vi "Controle_Manip_Main_GUI_Backup2.vi"() -> ()   [LabVIEW 2019] (continued)
                    n3203 = local write "Photodiode error out"(w3898) -> ()
                  }
                }
              }
            }
          }
          event "RotStage Exc Home", "RotStage Det Home", "Newport Linear Translation Stage Home": Mouse Down {
            n3204 = event-data() -> ("CtlRef"=w3923:refnum<vi>)  [unwired: 1 in, 7 out]
            n3205 = property class="Bool (strict)"(reference=w3923) -> ("Label.Text"=w3922:string)  [unwired: 1 in, 2 out]
            n3206 = case shown="\"Newport Linear Translation Stage Home\"" w3922 {
              tunnel: 0.0 -> [w3924 w3925 w3926]
              frame "RotStage Det Home", Default {
                n3207 = property on="RotStage Det Angle (°)" class="DigNum (strict)"("Val(Sgnl)"=w3924) -> ()  [unwired: 2 in, 2 out]
              }
              frame "Newport Linear Translation Stage Home" {
                n3208 = property on="Newport Linear Translation Stage Position (mm)" class="DigNum (strict)"("Val(Sgnl)"=w3925) -> ()  [unwired: 2 in, 2 out]
              }
              frame "RotStage Exc Home" {
                n3209 = property on="RotStage Exc Angle (°)" class="DigNum (strict)"("Val(Sgnl)"=w3926) -> ()  [unwired: 2 in, 2 out]
              }
            }
          }
          event "RotStage Exc Jog Backward", "RotStage Det Jog Backward", "RotStage Exc Jog Forward", "RotStage Det Jog Forward", "Newport Linear Translation Stage Jog Forward", "Newport Linear Translation Stage Jog Backward", "PZC Jog Forward", "PZC Jog Backward": Mouse Down {
            n3210 = event-data() -> ("CtlRef"=w3929:refnum<vi>)  [unwired: 1 in, 7 out]
            n3211 = property class="Bool (strict)"(reference=w3929) -> ("Label.Text"=w3927:string, "Value"=w3928:bool)  [unwired: 1 in, 2 out]
            n3212 = case shown="\"PZC Jog Backward\"" w3927 {
              tunnel: w3928 -> [_ _ _ _ _ _ _ _ _]
              frame "RotStage Det Jog Backward" {
                n3213 = local read "RotStage Det Angle Readout (°)"() -> (w3932:dbl)
                n3214 = local read "RotStage Det Angle Step (°)"() -> (w3931:dbl)
                n3215 = Subtract(x=w3932, y=w3931) -> (x-y=w3930:dbl)
                n3216 = property on="RotStage Det Angle (°)" class="DigNum (strict)"("Val(Sgnl)"=w3930) -> ()  [unwired: 2 in, 2 out]
              }
              frame "RotStage Det Jog Forward" {
                n3217 = local read "RotStage Det Angle Readout (°)"() -> (w3934:dbl)
                n3218 = local read "RotStage Det Angle Step (°)"() -> (w3935:dbl)
                n3219 = Add(x=w3934, y=w3935) -> (x+y=w3933:dbl)
                n3220 = property on="RotStage Det Angle (°)" class="DigNum (strict)"("Val(Sgnl)"=w3933) -> ()  [unwired: 2 in, 2 out]
              }
              frame "RotStage Exc Jog Forward" {
                n3221 = local read "RotStage Exc Angle Readout (°)"() -> (w3938:dbl)
                n3222 = local read "RotStage Exc Angle Step (°)"() -> (w3937:dbl)
                n3223 = Add(x=w3938, y=w3937) -> (x+y=w3936:dbl)
                n3224 = property on="RotStage Exc Angle (°)" class="DigNum (strict)"("Val(Sgnl)"=w3936) -> ()  [unwired: 2 in, 2 out]
              }
              frame "Newport Linear Translation Stage Jog Forward" {
                n3225 = local read "Newport Linear Translation Stage Position Readout (mm)"() -> (w3943:dbl)
                n3226 = local read "Newport Linear Translation Stage Step (mm)"() -> (w3942:dbl)
                n3227 = Add(x=w3943, y=w3942) -> (x+y=w3941:dbl)
                n3228 = property on="Newport Linear Translation Stage Position Readout (mm)" class="DigNum (strict)"() -> ("Maximum"=w3939:dbl)  [unwired: 2 in, 2 out]
                n3229 = Less Or Equal?(x=w3941, y=w3939) -> (x <= y?=w3940:bool)
                n3230 = case shown="True" w3940 {
                  tunnel: w3941 -> [_ w3947]
                  frame False {
                    n3231 = stacked-sequence {
                      frame #0 {
                        n3232 = property on="Newport Linear Translation Stage Position Readout (mm)" class="DigNum (strict)"("Blinking"=TRUE) -> ()  [unwired: 2 in, 2 out]
                      }
                      frame #1 {
                        n3233 = Wait (ms)(milliseconds to wait=u32 500) -> ()  [unwired: 1 out]
                      }
                      frame #2 {
                        n3234 = property on="Newport Linear Translation Stage Position Readout (mm)" class="DigNum (strict)"("Blinking"=FALSE) -> ()  [unwired: 2 in, 2 out]
                      }
                    }
                  }
                  frame True {
                    n3235 = property on="Newport Linear Translation Stage Position (mm)" class="DigNum (strict)"("Val(Sgnl)"=w3947) -> ()  [unwired: 2 in, 2 out]
                  }
                }
              }
              frame "Newport Linear Translation Stage Jog Backward" {
                n3236 = local read "Newport Linear Translation Stage Position Readout (mm)"() -> (w3952:dbl)
                n3237 = local read "Newport Linear Translation Stage Step (mm)"() -> (w3951:dbl)
                n3238 = Subtract(x=w3952, y=w3951) -> (x-y=w3949:dbl)
                n3239 = property on="Newport Linear Translation Stage Position Readout (mm)" class="DigNum (strict)"() -> ("Minimum"=w3948:dbl)  [unwired: 2 in, 2 out]
                n3240 = Greater Or Equal?(x=w3949, y=w3948) -> (x >= y?=w3950:bool)
                n3241 = case shown="False" w3950 {
                  tunnel: w3949 -> [_ w3956]
                  frame False {
                    n3242 = stacked-sequence {
                      frame #0 {
                        n3243 = property on="Newport Linear Translation Stage Position Readout (mm)" class="DigNum (strict)"("Blinking"=TRUE) -> ()  [unwired: 2 in, 2 out]
                      }
                      frame #1 {
                        n3244 = Wait (ms)(milliseconds to wait=u32 500) -> ()  [unwired: 1 out]
                      }
                      frame #2 {
                        n3245 = property on="Newport Linear Translation Stage Position Readout (mm)" class="DigNum (strict)"("Blinking"=FALSE) -> ()  [unwired: 2 in, 2 out]
                      }
                    }
                  }
                  frame True {
                    n3246 = property on="Newport Linear Translation Stage Position (mm)" class="DigNum (strict)"("Val(Sgnl)"=w3956) -> ()  [unwired: 2 in, 2 out]
                  }
                }
              }
              frame "RotStage Exc Jog Backward" {
                n3247 = local read "RotStage Exc Angle Readout (°)"() -> (w3959:dbl)
                n3248 = local read "RotStage Exc Angle Step (°)"() -> (w3958:dbl)
                n3249 = Subtract(x=w3959, y=w3958) -> (x-y=w3957:dbl)
                n3250 = property on="RotStage Exc Angle (°)" class="DigNum (strict)"("Val(Sgnl)"=w3957) -> ()  [unwired: 2 in, 2 out]
              }
              frame "PZC Jog Forward" {
                n3251 = local read "PZC200 Instrument Channel"() -> (w3977:string)
                n3252 = local read "PZC Speed (usteps/s)"() -> (w3968:u16)
                n3253 = Number To Decimal String(number=w3968) -> (decimal integer string=w3970:string)  [unwired: 1 in]
                n3254 = Concatenate Strings("1JA" ("Command"), w3970) -> (w3976:string)
                n3255 = call "SendCommand.vi"("Command"=w3976, "Instrument Channel"=w3977) -> ("error out"=w3974:errorcluster, "Instrument Channel out"=w3975:string)  [unwired: 8 in]
                n3256 = call "ReadCommand.vi"("Disable MAV check (F)"=FALSE, "error in"=w3974, "Instrument Channel"=w3975) -> ("error out"=w3971:errorcluster, "Instrument Channel out"=w3973:string)  [unwired: 6 in, 1 out]
                n3257 = while {
                  shift-right: [w3981] -> w3967
                  shift-left: w3973 -> [w3985]
                  shift-right: [w3979] -> w3966
                  shift-left: w3971 -> [w3980]
                  tunnel: ["1ST"] -> w3965
                  stop <- w3982 continue-if-true
                  n3258 = call "PZCGetPos.vi"("error in"=w3980, "Instrument Channel"=w3985) -> ("Instrument Channel Out"=w3981:string, "Position"=w3984:i32, "error out"=w3979:errorcluster)
                  n3259 = Wait (ms)(milliseconds to wait=u32 150) -> ()  [unwired: 1 out]
                  n3260 = local write "PZC Position Readout (usteps)"(w3984) -> ()
                  n3261 = local read "PZC Jog Forward"() -> (w3982:bool)
                }
                n3262 = call "SendCommand.vi"("error in"=w3966, "Command"=w3965, "Instrument Channel"=w3967) -> ("error out"=w3963:errorcluster, "Instrument Channel out"=w3964:string)  [unwired: 7 in]
                n3263 = call "PZCGetPos.vi"("error in"=w3963, "Instrument Channel"=w3964) -> ("Instrument Channel Out"=w3962:string, "Position"=w3960:i32, "error out"=w3961:errorcluster)
                n3264 = local write "PZC Position Readout (usteps)"(w3960) -> ()
                n3265 = local write "PZC Error"(w3961) -> ()
                n3266 = local write "PZC200 Instrument Channel"(w3962) -> ()
              }
              frame Default {
              }
              frame "PZC Jog Backward" {
                n3267 = local read "PZC Speed (usteps/s)"() -> (w3991:u16)
                n3268 = local read "PZC200 Instrument Channel"() -> (w4003:string)
                n3269 = Number To Decimal String(number=w3991) -> (decimal integer string=w3993:string)  [unwired: 1 in]
                n3270 = Concatenate Strings("1JA-" ("Command"), w3993) -> (w4002:string)
                n3271 = call "SendCommand.vi"("Command"=w4002, "Instrument Channel"=w4003) -> ("error out"=w4000:errorcluster, "Instrument Channel out"=w4001:string)  [unwired: 8 in]
                n3272 = call "ReadCommand.vi"("Disable MAV check (F)"=FALSE, "error in"=w4000, "Instrument Channel"=w4001) -> ("error out"=w3997:errorcluster, "Instrument Channel out"=w3998:string)  [unwired: 6 in, 1 out]
                n3273 = while {
                  shift-right: [w4005] -> w3996
                  shift-left: w3997 -> [w4006]
                  shift-right: [w4007] -> w3995
                  shift-left: w3998 -> [w4011]
                  tunnel: ["1ST"] -> w3994
                  stop <- w4009 continue-if-true
                  n3274 = call "PZCGetPos.vi"("error in"=w4006, "Instrument Channel"=w4011) -> ("Instrument Channel Out"=w4007:string, "Position"=w4010:i32, "error out"=w4005:errorcluster)
                  n3275 = Wait (ms)(milliseconds to wait=u32 150) -> ()  [unwired: 1 out]
                  n3276 = local write "PZC Position Readout (usteps)"(w4010) -> ()
                  n3277 = local read "PZC Jog Backward"() -> (w4009:bool)
                }
                n3278 = call "SendCommand.vi"("error in"=w3996, "Command"=w3994, "Instrument Channel"=w3995) -> ("error out"=w3990:errorcluster, "Instrument Channel out"=w3989:string)  [unwired: 7 in]
                n3279 = call "PZCGetPos.vi"("error in"=w3990, "Instrument Channel"=w3989) -> ("Instrument Channel Out"=w3988:string, "Position"=w3986:i32, "error out"=w3987:errorcluster)
                n3280 = local write "PZC Position Readout (usteps)"(w3986) -> ()
                n3281 = local write "PZC Error"(w3987) -> ()
                n3282 = local write "PZC200 Instrument Channel"(w3988) -> ()
              }
            }
          }
          event "RotStage Exc Velocity (°/s)", "RotStage Det Velocity (°/s)", "Newport Linear Translation Stage Velocity (mm/s)": Value Change {
            n3283 = event-data() -> ("CtlRef"=w4014:refnum<vi>, "NewVal"=w4013:dbl)  [unwired: 1 in, 4 out]
            n3284 = local read "ESP 301 On?"() -> (w4012:bool)
            n3285 = case shown="True" w4012 {
              tunnel: w4014 -> [_ w4021]
              tunnel: w4013 -> [_ w4019]
              frame False {
              }
              frame True {
                n3286 = local read "ESP 301 COM Port"() -> (w4018:refnum<visa-resource-name>)
                n3287 = property class="DigNum (strict)"(reference=w4021) -> ("Label.Text"=w4020:string)  [unwired: 1 in, 2 out]
                n3288 = local read "ESP 301 Error"() -> (w4017:errorcluster)
                n3289 = case shown="\"RotStage Det Velocity (°/s)\"" w4020 {
                  tunnel: w4019 -> [w4025 _ w4030 w4040]
                  tunnel: w4018 -> [w4026 w4029 w4032 w4039]
                  tunnel: w4017 -> [w4027 w4028 w4033 w4038]
                  tunnel: [w4023 w4029 w4035 w4037] -> w4016
                  tunnel: [w4022 w4028 w4034 w4036] -> w4015
                  frame "Newport Linear Translation Stage Velocity (mm/s)" {
                    n3290 = call "Set Velocity.vi"("error in (no error)"=w4027, "Velocity (units/s)"=w4025, "Axis (1)"=1, "VISA resource name"=w4026) -> ("error out"=w4022:errorcluster, "VISA resource name out"=w4023:refnum<visa-resource-name>)  [unwired: 2 in]
                  }
                  frame Default {
                  }
                  frame "RotStage Det Velocity (°/s)" {
                    n3291 = call "Set Velocity.vi"("error in (no error)"=w4033, "Velocity (units/s)"=w4030, "Axis (1)"=2, "VISA resource name"=w4032) -> ("error out"=w4034:errorcluster, "VISA resource name out"=w4035:refnum<visa-resource-name>)  [unwired: 2 in]
                  }
                  frame "RotStage Exc Velocity (°/s)" {
                    n3292 = call "Set Velocity.vi"("error in (no error)"=w4038, "Velocity (units/s)"=w4040, "Axis (1)"=3, "VISA resource name"=w4039) -> ("error out"=w4036:errorcluster, "VISA resource name out"=w4037:refnum<visa-resource-name>)  [unwired: 2 in]
                  }
                }
                n3293 = local write "ESP 301 COM Port"(w4016) -> ()
                n3294 = local write "ESP 301 Error"(w4015) -> ()
              }
            }
          }
          event "Save Spectrum", "Save Spectrum N", "Save XY Map", "Save Polarisation", "Save Contrast", "Save Michelson", "Save Custom Diode Spectrum", "Save fPow", "Save PLE": Value Change {
            n3295 = event-data() -> ("CtlRef"=w4049:refnum<vi>)  [unwired: 1 in, 3 out]
            n3296 = property class="Bool (strict)"(reference=w4049) -> ("Label.Text"=w4048:string)  [unwired: 1 in, 2 out]
            n3297 = stacked-sequence {
              tunnel: w4048 -> [_ w4098 _]
              tunnel: [_ w4095 _] -> w4046
              tunnel: [_ w4097 _] -> w4047
              tunnel: [_ w4092 _] -> w4044
              tunnel: [w4050 _ _] -> w4043
              tunnel: [_ w4093 _] -> w4045
              frame #0 {
                n3298 = local read "Excitation Wavelength (nm)"() -> (w4072:dbl)
                n3299 = local read "Wavelength calibration"() -> (w4073:dbl[])
                n3300 = local read "Center Wavelength (nm)"() -> (w4081:dbl)
                n3301 = local read "Experiment Name With Date"() -> (w4077:string)
                n3302 = local read "Map Marker Y Pos"() -> (w4063:i8)
                n3303 = local read "Scan Y Readout (V)"() -> (w4061:dbl)
                n3304 = local read "Scan X Readout (V)"() -> (w4062:dbl)
                n3305 = local read "Exposure Time (ms)"() -> (w4074:dbl)
                n3306 = local read "Map Marker X Pos"() -> (w4064:i8)
                n3307 = local read "Exposure Time (ms)"() -> (w4078:dbl)
                n3308 = local read "Attocubes On?"() -> (w4068:bool)
                n3309 = local read "Excitation Source"() -> (w4079:enum16{"P", "CW", "SK"})
                n3310 = local read "Temperature (K)"() -> (w4082:dbl)
                n3311 = local read "Excitation Power (uW)"() -> (w4084:dbl)
                n3312 = local read "Comment"() -> (w4083:string)
                n3313 = local read "Acq Mode"() -> (w4076:T3)
                n3314 = local read "Log file"() -> (w4075:string)
                n3315 = case shown="True" w4068 {
                  tunnel: [w4085 w4088] -> w4067
                  tunnel: [w4085 w4087] -> w4066
                  tunnel: [w4085 w4086] -> w4065
                  frame False {
                    w4085 = nan
                  }
                  frame True {
                    n3316 = local read "Att Pos Y"() -> (w4087:dbl)
                    n3317 = local read "Att Pos X"() -> (w4088:dbl)
                    n3318 = local read "Att Pos Z"() -> (w4086:dbl)
                  }
                }
                n3319 = Multiply(x=w4084, y=1000000.0) -> (x*y=w4080:dbl)
                n3320 = local read "LightField On?"() -> (w4070:bool)
                n3321 = Bundle("Att Pos X"=w4067, "Att Pos Y"=w4066, "Att Pos Z"=w4065, "Map Marker X Pos"=w4064, "Map Marker Y Pos"=w4063, "Scan X Readout (V)"=w4062, "Scan Y Readout (V)"=w4061) -> (w4060:T5)  [unwired: 1 in]
                "Location cluster" <- w4060
                n3322 = case shown="False" w4070 {
                  tunnel: ["" w4090] -> w4069
                  frame False {
                  }
                  frame True {
                    n3323 = local read "Grating"() -> (w4090:string)
                  }
                }
                n3324 = Bundle("Sample first cooldown"="Sample first cooldown", "SampleOf"="SampleOf", "Synthesis/Name"="Synthesis/Name", "Synthesis/InjTemp"="Synthesis/InjTemp", "Synthesis/Dilution"="Synthesis/Dilution", "Synthesis/Polymer"="Synthesis/Polymer", "Synthesis/DilutionPolyRatio"="Synthesis/DilutionPolyRatio", "Synthesis/Solvent"="Synthesis/Solvent") -> (w4051:T40)  [unwired: 1 in]
                n3325 = Bundle("Comment"=w4083, "Temperature (K)"=w4082, "Center Wavelength (nm)"=w4081, w4080, "Excitation Source"=w4079, "Exposure Time (ms)"=w4078, "Experiment Name With Date"=w4077, "Acq Mode"=w4076, "Log file"=w4075, "Exposure Time (ms)"=w4074, "Wavelength calibration"=w4073, "Excitation Wavelength (nm)"=w4072, "Grating"=w4069, w4060, w4051) -> (w4050:T41)  [unwired: 1 in]
                "Params Save" <- w4050
              }
              frame #1 {
                n3326 = case shown="\"Save Contrast\"" w4098 {
                  tunnel: [w4102 w4147 w4172 w4196 w4218 w4248 w4271 w4294 w4343] -> w4095
                  tunnel: [w4101 w4145 w4171 w4195 w4217 w4247 w4270 w4293 w4340] -> w4092
                  tunnel: [w4100 w4146 w4170 w4194 w4216 w4246 w4269 w4292 w4334] -> w4096
                  tunnel: [w4099 w4144 w4169 w4193 w4215 w4245 w4268 w4291 w4333] -> w4093
                  frame "Save Spectrum N" {
                    n3327 = local read "Acq Mode"() -> (w4103:T3)
                    n3328 = case shown="\"Spectrum\", Default" w4103 {
                      tunnel: [w4112 w4133] -> w4102
                      tunnel: [w4111 w4132] -> w4101
                      tunnel: [w4105 w4126] -> w4100
                      tunnel: [w4104 w4125] -> w4099
                      frame "Spectrum", Default {
                        w4104 = T42."Time Trace" ("Measurement type")
                        n3329 = invoke on="CCD 2D Image Main" class="IntGraph (strict)" method="Get Image"() -> ("image data"=w4105:T43)  [unwired: 6 in, 5 out]
                        n3330 = local read "BackgroundSpec"() -> (w4109:dbl[])
                        n3331 = local read "Pol in path?"() -> (w4108:bool)
                        n3332 = local read "DotNum"() -> (w4110:dbl)
                        n3333 = local read "Data"() -> (w4118:T26)
                        n3334 = local read "Params Save"() -> (w4121:T4)
                        n3335 = Index Array(array=w4118, index=0) -> (element=w4116:T44)
                        n3336 = case shown="True" w4108 {
                          tunnel: [w4122 w4123] -> w4106
                          tunnel: [w4122 w4124] -> w4107
                          frame False {
                            w4122 = nan
                          }
                          frame True {
                            n3337 = local read "RotStage Exc Angle Readout (°)"() -> (w4124:dbl)
                            n3338 = local read "RotStage Det Angle Readout (°)"() -> (w4123:dbl)
                          }
                        }
                        n3339 = Unbundle By Name(w4116) -> ("Image"=w4115:dbl[][][])
                        "Image" <- w4115
                        n3340 = Index Array(array=w4115, index (dim 1)=0 ("disabled index (row)")) -> (element=w4114:dbl[][])  [unwired: 2 in]
                        n3341 = Build Array(w4107) -> (w4120:dbl[])
                        n3342 = Build Array(w4106) -> (w4119:dbl[])
                        n3343 = call "Format&SaveDataCleanbckp.vi"("Measurement type"=w4104, "Params Save"=w4121, "DotNum"=w4110, "Suppl"=w4109, "Data_CCD_px"=w4114, "L2Exc_deg"=w4120, "L2Det_deg"=w4119) -> ("FullComment"=w4111:string, "WrittenDatasetName"=w4112:string)  [unwired: 9 in, 2 out]
                      }
                      frame "Image" {
                        w4125 = T42."Time Trace" ("Measurement type")
                        n3344 = invoke on="CCD 2D Image Main" class="IntGraph (strict)" method="Get Image"() -> ("image data"=w4126:T43)  [unwired: 6 in, 5 out]
                        n3345 = local read "BackgroundSpec"() -> (w4130:dbl[])
                        n3346 = local read "Pol in path?"() -> (w4129:bool)
                        n3347 = local read "DotNum"() -> (w4131:dbl)
                        n3348 = local read "Data"() -> (w4137:T26)
                        n3349 = local read "Params Save"() -> (w4140:T4)
                        n3350 = case shown="True" w4129 {
                          tunnel: [w4141 w4142] -> w4127
                          tunnel: [w4141 w4143] -> w4128
                          frame False {
                            w4141 = nan
                          }
                          frame True {
                            n3351 = local read "RotStage Exc Angle Readout (°)"() -> (w4143:dbl)
                            n3352 = local read "RotStage Det Angle Readout (°)"() -> (w4142:dbl)
                          }
                        }
                        n3353 = Index Array(array=w4137, index=0) -> (element=w4135:T44)
                        n3354 = Unbundle By Name(w4135) -> ("Image"=w4134:dbl[][][])
                        n3355 = Build Array(w4128) -> (w4139:dbl[])
                        n3356 = Build Array(w4127) -> (w4138:dbl[])
                        n3357 = call "Format&SaveDataCleanbckp.vi"("Measurement type"=w4125, "Params Save"=w4140, "DotNum"=w4131, "Main 3D Data to write"=w4134, "Suppl"=w4130, "L2Exc_deg"=w4139, "L2Det_deg"=w4138) -> ("FullComment"=w4132:string, "WrittenDatasetName"=w4133:string)  [unwired: 9 in, 2 out]
                      }
                    }
                  }
                  frame "Save XY Map" {
                    w4144 = T42."XY Intensity Map" ("Measurement type")
                    n3358 = local read "Pol in path?"() -> (w4158:bool)
                    n3359 = local read "Params Save"() -> (w4165:T4)
                    n3360 = local read "BackgroundSpec"() -> (w4162:dbl[])
                    n3361 = local read "Params XY Map SubVI"() -> (w4155:T23)
                    n3362 = local read "Map Marker Y Pos"() -> (w4153:i8)
                    n3363 = local read "XYMap Data"() -> (w4164:i32[][])
                    n3364 = local read "Map Marker X Pos"() -> (w4154:i8)
                    n3365 = local read "XYPositions"() -> (w4161:dbl[][])
                    n3366 = Format Into String(w4154) -> (resulting string=w4152:string)  [unwired: 3 in, 1 out]
                    n3367 = Format Into String(w4153) -> (resulting string=w4151:string)  [unwired: 3 in, 1 out]
                    n3368 = case shown="True" w4158 {
                      tunnel: [w4166 w4167] -> w4157
                      tunnel: [w4166 w4168] -> w4156
                      frame False {
                        w4166 = nan
                      }
                      frame True {
                        n3369 = local read "RotStage Exc Angle Readout (°)"() -> (w4168:dbl)
                        n3370 = local read "RotStage Det Angle Readout (°)"() -> (w4167:dbl)
                      }
                    }
                    n3371 = Concatenate Strings("\n### Map @ " ("string"), w4152, "x" ("string"), w4151) -> (w4150:string)
                    n3372 = call "Write2Markdown.vi"("String"=w4150) -> ()
                    n3373 = disable-structure shown="Disabled" {
                      frame Disabled {
                        n3374 = local read "XYPos Indices"() -> ()  [unwired: 1 out]
                      }
                      frame Enabled {
                      }
                    }
                    n3375 = Build Array(w4157) -> (w4160:dbl[])
                    n3376 = Build Array(w4156) -> (w4159:dbl[])
                    n3377 = call "Format&SaveDataCleanbckp.vi"("Measurement type"=w4144, "Suppl_2D"=w4161, "Params Save"=w4165, "DotNum"=0.0, "Params XY Map SubVI"=w4155, "Suppl"=w4162, "Data_CCD_px"=w4164, "L2Exc_deg"=w4159, "L2Det_deg"=w4160) -> ("FullComment"=w4145:string, "WrittenDatasetName"=w4147:string)  [unwired: 7 in, 2 out]
                    n3378 = invoke on="XY Intensity Map" class="IntGraph (strict)" method="Get Image"() -> ("image data"=w4146:T43)  [unwired: 6 in, 5 out]
                  }
                  frame "Save Contrast" {
                    n3379 = local read "Acq Mode"() -> (w4173:T3)
                    n3380 = case shown="\"Spectrum\", Default" w4173 {
                      tunnel: [w4183] -> w4172
                      tunnel: [w4182] -> w4171
                      tunnel: [w4176] -> w4170
                      tunnel: [w4175] -> _
                      tunnel: [w4174] -> w4169
                      frame "Spectrum", Default {
                        w4174 = T42."Contrast" ("Measurement type")
                        n3381 = invoke on="Contrast Oscillations" class="XYGraph (strict)" method="Get Image"() -> ("image data"=w4176:T43)  [unwired: 6 in, 5 out]
                        n3382 = local read "Pol in path?"() -> (w4179:bool)
                        n3383 = local read "BackgroundSpec"() -> (w4180:dbl[])
                        n3384 = local read "DotNum"() -> (w4181:dbl)
                        n3385 = local read "Params Save"() -> (w4189:T4)
                        n3386 = case shown="True" w4179 {
                          tunnel: [w4190 w4191] -> w4177
                          tunnel: [w4190 w4192] -> w4178
                          frame False {
                            w4190 = nan
                          }
                          frame True {
                            n3387 = local read "RotStage Exc Angle Readout (°)"() -> (w4192:dbl)
                            n3388 = local read "RotStage Det Angle Readout (°)"() -> (w4191:dbl)
                          }
                        }
                        n3389 = local read "Contrast Array Out"() -> (w4186:dbl[][])
                        n3390 = local read "PZAPos&Pow"() -> (w4184:dbl[][])
                        n3391 = Build Array(w4178) -> (w4188:dbl[])
                        n3392 = Build Array(w4177) -> (w4187:dbl[])
                        n3393 = Transpose 2D Array(2D array=w4186) -> (transposed array=w4185:dbl[][])
                        n3394 = call "Format&SaveDataCleanbckp.vi"("Measurement type"=w4174, "Suppl_2D"=w4184, "Params Save"=w4189, "DotNum"=w4181, "Suppl"=w4180, "Data_CCD_px"=w4185, "L2Exc_deg"=w4188, "L2Det_deg"=w4187) -> ("datasetnumber"=w4175:string, "FullComment"=w4182:string, "WrittenDatasetName"=w4183:string)  [unwired: 8 in, 1 out]
                      }
                    }
                  }
                  frame "Save Michelson" {
                    n3395 = local read "Acq Mode"() -> (w4197:T3)
                    n3396 = case shown="\"Spectrum\", Default" w4197 {
                      tunnel: [w4206] -> w4196
                      tunnel: [w4205] -> w4195
                      tunnel: [w4199] -> w4194
                      tunnel: [w4198] -> w4193
                      frame "Spectrum", Default {
                        w4198 = T42."Michelson" ("Measurement type")
                        n3397 = local read "BackgroundSpec"() -> (w4203:dbl[])
                        n3398 = invoke on="Contrast Oscillations" class="XYGraph (strict)" method="Get Image"() -> ("image data"=w4199:T43)  [unwired: 6 in, 5 out]
                        n3399 = local read "Pol in path?"() -> (w4202:bool)
                        n3400 = local read "DotNum"() -> (w4204:dbl)
                        n3401 = local read "Params Save"() -> (w4211:T4)
                        n3402 = case shown="True" w4202 {
                          tunnel: [w4212 w4213] -> w4200
                          tunnel: [w4212 w4214] -> w4201
                          frame False {
                            w4212 = nan
                          }
                          frame True {
                            n3403 = local read "RotStage Exc Angle Readout (°)"() -> (w4214:dbl)
                            n3404 = local read "RotStage Det Angle Readout (°)"() -> (w4213:dbl)
                          }
                        }
                        n3405 = local read "Michelson Array Out"() -> (w4207:dbl[][][])
                        n3406 = local read "PZC&Pow3D"() -> (w4208:dbl[][][])
                        n3407 = Build Array(w4201) -> (w4210:dbl[])
                        n3408 = Build Array(w4200) -> (w4209:dbl[])
                        n3409 = call "Format&SaveDataCleanbckp.vi"("Measurement type"=w4198, "Params Save"=w4211, "DotNum"=w4204, "Main 3D Data to write"=w4207, "Suppl"=w4203, "L2Exc_deg"=w4210, "L2Det_deg"=w4209, "Suppl_3D"=w4208) -> ("FullComment"=w4205:string, "WrittenDatasetName"=w4206:string)  [unwired: 8 in, 2 out]
                      }
                    }
                  }
                  frame "Save Polarisation" {
                    n3410 = local read "Acq Mode"() -> (w4219:T3)
                    n3411 = case shown="\"Spectrum\", Default" w4219 {
                      tunnel: [w4229] -> w4218
                      tunnel: [w4228] -> w4217
                      tunnel: [w4222] -> w4216
                      tunnel: [w4221] -> w4215
                      frame "Spectrum", Default {
                        w4221 = T42."Polarisation" ("Measurement type")
                        n3412 = local read "Pol in path?"() -> (w4225:bool)
                        n3413 = case shown="True" w4225 {
                          tunnel: [w4232 w4235] -> w4224
                          tunnel: [w4232 w4234] -> w4223
                          frame False {
                            n3414 = Build Array(nan) -> (w4232:dbl[])
                          }
                          frame True {
                            n3415 = local read "Polar mode"() -> (w4236:u16)
                            n3416 = case shown="3, Default" w4236 {
                              tunnel: [w4238 w4240] -> w4235
                              tunnel: [w4237 w4243] -> w4234
                              frame 2 {
                                n3417 = local read "RotStage Exc Angle Readout (°)"() -> (w4239:dbl)
                                n3418 = local read "Angles"() -> (w4237:dbl[])
                                n3419 = Build Array(w4239) -> (w4238:dbl[])
                              }
                              frame 3, Default {
                                n3420 = local read "PuissancesPolar"() -> (w4241:dbl[])
                                n3421 = local read "Angles"() -> (w4242:dbl[])
                                n3422 = local read "RotStage Det Angle Readout (°)"() -> (w4244:dbl)
                                n3423 = Insert Into Array(array=w4242, new element=w4241) -> (w4240:dbl[])  [unwired: 1 in]
                                n3424 = Build Array(w4244) -> (w4243:dbl[])
                              }
                            }
                          }
                        }
                        n3425 = local read "PuissancesPolar"() -> (w4220:dbl[])
                        n3426 = local read "BackgroundSpec"() -> (w4226:dbl[])
                        n3427 = local read "Params Save"() -> (w4231:T4)
                        n3428 = local read "DotNum"() -> (w4227:dbl)
                        n3429 = invoke on="Polarisation 2D Image" class="IntGraph (strict)" method="Get Image"() -> ("image data"=w4222:T43)  [unwired: 6 in, 5 out]
                        n3430 = property on="Polarisation 2D Image" class="IntGraph (strict)"() -> ("Value"=w4230:dbl[][])  [unwired: 2 in, 2 out]
                        n3431 = call "Format&SaveDataCleanbckp.vi"("Data_Angle_deg"=w4220, "Measurement type"=w4221, "Params Save"=w4231, "DotNum"=w4227, "Suppl"=w4226, "Data_CCD_px"=w4230, "L2Exc_deg"=w4224, "L2Det_deg"=w4223) -> ("FullComment"=w4228:string, "WrittenDatasetName"=w4229:string)  [unwired: 8 in, 2 out]
                      }
                    }
                  }
                  frame "Save PLE" {
                    n3432 = local read "Acq Mode"() -> (w4249:T3)
                    n3433 = case shown="\"Spectrum\", Default" w4249 {
                      tunnel: [w4260] -> w4248
                      tunnel: [w4259] -> w4247
                      tunnel: [w4250] -> w4246
                      tunnel: [w4253] -> w4245
                      frame "Spectrum", Default {
                        w4253 = T45."PLE" ("Measurement type")
                        n3434 = local read "Pol in path?"() -> (w4257:bool)
                        n3435 = local read "PLE 2D ExcWL&Pow"() -> (w4252:dbl[][])
                        n3436 = local read "PLE Raw Intensity"() -> (w4251:i32[][])
                        n3437 = case shown="True" w4257 {
                          tunnel: [w4262 w4267] -> w4255
                          tunnel: [w4262 w4264] -> w4254
                          frame False {
                            n3438 = Build Array(nan) -> (w4262:dbl[])
                          }
                          frame True {
                            n3439 = local read "RotStage Exc Angle Readout (°)"() -> (w4266:dbl)
                            n3440 = local read "RotStage Det Angle Readout (°)"() -> (w4265:dbl)
                            n3441 = Build Array(w4266) -> (w4267:dbl[])
                            n3442 = Build Array(w4265) -> (w4264:dbl[])
                          }
                        }
                        n3443 = local read "BackgroundSpec"() -> (w4256:dbl[])
                        n3444 = local read "Params Save"() -> (w4261:T4)
                        n3445 = local read "DotNum"() -> (w4258:dbl)
                        n3446 = call "Format&SaveDataCleanbckp.vi"("Measurement type"=w4253, "Suppl_2D"=w4252, "Params Save"=w4261, "DotNum"=w4258, "Suppl"=w4256, "Data_CCD_px"=w4251, "L2Exc_deg"=w4255, "L2Det_deg"=w4254) -> ("FullComment"=w4259:string, "WrittenDatasetName"=w4260:string)  [unwired: 8 in, 2 out]
                        n3447 = invoke on="PLE Raw Intensity" class="IntGraph (strict)" method="Get Image"() -> ("image data"=w4250:T43)  [unwired: 6 in, 5 out]
                      }
                    }
                  }
                  frame "Save fPow" {
                    n3448 = local read "Acq Mode"() -> (w4272:T3)
                    n3449 = case shown="\"Spectrum\", Default" w4272 {
                      tunnel: [w4285] -> w4271
                      tunnel: [w4284] -> w4270
                      tunnel: [w4273] -> w4269
                      tunnel: [w4276] -> w4268
                      frame "Spectrum", Default {
                        w4276 = T42."fPow" ("Measurement type")
                        n3450 = local read "DotNum"() -> (w4282:dbl)
                        n3451 = local read "Pol in path?"() -> (w4279:bool)
                        n3452 = local read "Array fPow Pow"() -> (w4275:dbl[])
                        n3453 = local read "Params Save"() -> (w4280:T4)
                        n3454 = case shown="False" w4279 {
                          tunnel: [w4288 w4290] -> w4278
                          tunnel: [w4288 w4289] -> w4277
                          frame False {
                            w4288 = nan
                          }
                          frame True {
                            n3455 = local read "RotStage Exc Angle Readout (°)"() -> (w4289:dbl)
                            n3456 = local read "RotStage Det Angle Readout (°)"() -> (w4290:dbl)
                          }
                        }
                        n3457 = local read "Array fPow"() -> (w4283:i32[][])
                        n3458 = Build Array(w4275, w4275) -> (w4274:dbl[][])
                        n3459 = invoke on="CCD 2D Image Main" class="IntGraph (strict)" method="Get Image"() -> ("image data"=w4273:T43)  [unwired: 6 in, 5 out]
                        n3460 = local read "BackgroundSpec"() -> (w4281:dbl[])
                        n3461 = Build Array(w4277) -> (w4287:dbl[])
                        n3462 = Build Array(w4278) -> (w4286:dbl[])
                        n3463 = call "Format&SaveDataCleanbckp.vi"("Measurement type"=w4276, "Suppl_2D"=w4274, "Params Save"=w4280, "DotNum"=w4282, "Suppl"=w4281, "Data_CCD_px"=w4283, "L2Exc_deg"=w4287, "L2Det_deg"=w4286) -> ("FullComment"=w4284:string, "WrittenDatasetName"=w4285:string)  [unwired: 8 in, 2 out]
                      }
                    }
                  }
                  frame "Save Spectrum", Default {
                    n3464 = local read "Acq Mode"() -> (w4295:T3)
                    n3465 = case shown="\"Spectrum\", Default" w4295 {
                      tunnel: [w4304 w4316] -> w4294
                      tunnel: [w4303 w4323] -> w4293
                      tunnel: [w4297 w4317] -> w4292
                      tunnel: [w4296 w4315] -> w4291
                      frame "Spectrum", Default {
                        w4296 = T42."Spectrum" ("Measurement type")
                        n3466 = local read "Pol in path?"() -> (w4300:bool)
                        n3467 = invoke on="CCD 1D Spectrum Main" class="XYGraph (strict)" method="Get Image"() -> ("image data"=w4297:T43)  [unwired: 6 in, 5 out]
                        n3468 = local read "CCD 1D Spectrum Main"() -> (w4308:cluster{dbl[], dbl[]})
                        n3469 = local read "DotNum"() -> (w4302:dbl)
                        n3470 = local read "BackgroundSpec"() -> (w4301:dbl[])
                        n3471 = local read "Params Save"() -> (w4311:T4)
                        n3472 = case shown="True" w4300 {
                          tunnel: [w4312 w4313] -> w4298
                          tunnel: [w4312 w4314] -> w4299
                          frame False {
                            w4312 = nan
                          }
                          frame True {
                            n3473 = local read "RotStage Exc Angle Readout (°)"() -> (w4314:dbl)
                            n3474 = local read "RotStage Det Angle Readout (°)"() -> (w4313:dbl)
                          }
                        }
                        n3475 = Unbundle(w4308) -> (w4307:dbl[], w4306:dbl[])
                        n3476 = Build Array(w4299) -> (w4310:dbl[])
                        n3477 = Build Array(w4298) -> (w4309:dbl[])
                        n3478 = Build Array(w4307, w4306) -> (w4305:dbl[][])
                        n3479 = call "Format&SaveDataCleanbckp.vi"("Measurement type"=w4296, "Params Save"=w4311, "DotNum"=w4302, "Suppl"=w4301, "Data_CCD_px"=w4305, "L2Exc_deg"=w4310, "L2Det_deg"=w4309) -> ("FullComment"=w4303:string, "WrittenDatasetName"=w4304:string)  [unwired: 9 in, 2 out]
                      }
                      frame "Image" {
                        w4315 = T42."Spectrum" ("Measurement type")
                        n3480 = invoke on="CCD 2D Image Main" class="IntGraph (strict)" method="Get Image"() -> ("image data"=w4317:T43)  [unwired: 6 in, 5 out]
                        n3481 = local read "BackgroundSpec"() -> (w4321:dbl[])
                        n3482 = local read "Pol in path?"() -> (w4320:bool)
                        n3483 = local read "DotNum"() -> (w4322:dbl)
                        n3484 = local read "Data"() -> (w4326:T26)
                        n3485 = case shown="True" w4320 {
                          tunnel: [w4330 w4331] -> w4318
                          tunnel: [w4330 w4332] -> w4319
                          frame False {
                            w4330 = nan
                          }
                          frame True {
                            n3486 = local read "RotStage Exc Angle Readout (°)"() -> (w4332:dbl)
                            n3487 = local read "RotStage Det Angle Readout (°)"() -> (w4331:dbl)
                          }
                        }
                        n3488 = Index Array(array=w4326) -> (element=w4325:T44)  [unwired: 1 in]
                        n3489 = Unbundle By Name(w4325) -> ("Image"=w4324:dbl[][][])
                        n3490 = local read "Params Save"() -> (w4329:T4)
                        n3491 = Build Array(w4319) -> (w4328:dbl[])
                        n3492 = Build Array(w4318) -> (w4327:dbl[])
                        n3493 = call "Format&SaveDataCleanbckp.vi"("Measurement type"=w4315, "Params Save"=w4329, "DotNum"=w4322, "Main 3D Data to write"=w4324, "Suppl"=w4321, "L2Exc_deg"=w4328, "L2Det_deg"=w4327) -> ("FullComment"=w4323:string, "WrittenDatasetName"=w4316:string)  [unwired: 9 in, 2 out]
                      }
                    }
                  }
                  frame "Save Custom Diode Spectrum" {
                    w4333 = T42."Spectrum" ("Measurement type")
                    n3494 = local read "Spectrum Custom Mode"() -> (w4339:u16)
                    n3495 = local read "Data PL Custom Diode Spectrum"() -> (w4346:dbl[])
                    n3496 = local read "DotNum"() -> (w4338:dbl)
                    n3497 = local read "Params Save"() -> (w4347:T4)
                    n3498 = local read "Pol in path?"() -> (w4337:bool)
                    n3499 = invoke on="CCD 1D Spectrum Main" class="XYGraph (strict)" method="Get Image"() -> ("image data"=w4334:T43)  [unwired: 6 in, 5 out]
                    n3500 = local read "Wavelength calibration"() -> (w4345:dbl[])
                    n3501 = case shown="True" w4337 {
                      tunnel: [w4348 w4349] -> w4335
                      tunnel: [w4348 w4350] -> w4336
                      frame False {
                        w4348 = nan
                      }
                      frame True {
                        n3502 = local read "RotStage Exc Angle Readout (°)"() -> (w4350:dbl)
                        n3503 = local read "RotStage Det Angle Readout (°)"() -> (w4349:dbl)
                      }
                    }
                    n3504 = Build Array(w4345, w4346) -> (w4344:dbl[][])
                    n3505 = Build Array(w4336) -> (w4342:dbl[])
                    n3506 = Build Array(w4335) -> (w4341:dbl[])
                    n3507 = call "Format&SaveDataCleanbckp.vi"("Measurement type"=w4333, "Spectrum Custom Mode"=w4339, "Params Save"=w4347, "DotNum"=w4338, "Data_CCD_px"=w4344, "L2Exc_deg"=w4342, "L2Det_deg"=w4341) -> ("FullComment"=w4340:string, "WrittenDatasetName"=w4343:string)  [unwired: 9 in, 2 out]
                  }
                }
                "WrittenDatasetName" <- w4095
                "FullComment" <- w4092
                n3508 = local read "Params Save"() -> (w4091:T4)
                n3509 = call "AutoScreenShot.vi"("Params Save"=w4091, "Figure image data"=w4096, "Datasetname"=w4095) -> ("imagefilename"=→"imagefilename":string)  [unwired: 1 in]
                n3510 = local read "Log file"() -> (w4097:string)
              }
              frame #2 {
                w4353 = FALSE
                n3511 = local write "Comment"("") -> ()
                n3512 = local write "Save Custom Diode Spectrum"(w4353) -> ()
                n3513 = local write "Save Michelson"(w4353) -> ()
                n3514 = local write "Save Contrast"(w4353) -> ()
                n3515 = local write "Save XY Map"(w4353) -> ()
                n3516 = local write "Save Spectrum"(w4353) -> ()
                n3517 = local write "Save Polarisation"(w4353) -> ()
                n3518 = local write "Save Spectrum N"(w4353) -> ()
                n3519 = local write "Save fPow"(w4353) -> ()
                n3520 = local read "DotNum"() -> (→"LastDotNum":dbl)
              }
            }
            n3521 = call "WriteSave2MarkdownWithImages.vi"("Measurement type"=w4045, "Full Comment"=w4044, "Params Save"=w4043, "Written Dataset Name"=w4046, "Log file"=w4047) -> ("Log file after"=w4042:string)  [unwired: 1 in]
            n3522 = local write "Log file"(w4042) -> ()
          }
          event "Connect": Value Change {
            n3523 = event-data() -> ("NewVal"=w4354:bool)  [unwired: 1 in, 5 out]
            n3524 = case shown="False" w4354 {
              frame False {
                n3525 = local read "PH_Init_Data"() -> (w4357:T11)
                n3526 = Unbundle By Name(w4357) -> ("Deviceindex"=w4356:i32)
                n3527 = local write "Connected"(FALSE) -> ()
                n3528 = call "PH_Close.vi"("devidx"=w4356) -> ()
              }
              frame True {
                n3529 = local read "PicoHarp On?"() -> (w4358:bool)
                n3530 = case shown="True" w4358 {
                  frame False {
                  }
                  frame True {
                    n3531 = local read "Log file"() -> (w4360:string)
                    n3532 = property on="Experiment Graph Controls" class="TabCtl (strict)"("Value"=T25."APDs" ("Experiment Graph Controls")) -> ("Pages"=w4365:refnum<vi>[])  [unwired: 2 in, 2 out]
                    n3533 = call "Write2LogFile.vi"("Add to log file"="Initialise communication with PicoHarp", "Log file before"=w4360, "Checkbox"=FALSE) -> ("Log file after"=w4361:string)
                    n3534 = call "PH_Init.vi"() -> ("PH_Init_Data"=w4359:T11)
                    n3535 = local write "Log file"(w4361) -> ()
                    n3536 = Index Array(array=w4365, index=4) -> (element=w4364:refnum<vi>)
                    n3537 = property class="Page"(reference=w4364, "PageVis"=TRUE ("Page Visible")) -> ()  [unwired: 1 in, 2 out]
                    n3538 = local write "PH_Init_Data"(w4359) -> ()
                    n3539 = local write "Connected"(TRUE) -> ()
                  }
                }
              }
            }
          }
          event "ChangeSample": Mouse Down {
            n3540 = event-data() -> ()  [unwired: 1 in, 8 out]
            n3541 = local read "Synthesis/DilutionPolyRatio"() -> (w4380:dbl)
            n3542 = local read "Synthesis/Polymer"() -> (w4383:string)
            n3543 = local read "Synthesis/Solvent"() -> (w4382:string)
            n3544 = local read "Sample first cooldown"() -> (w4384:timestamp)
            n3545 = local read "Synthesis/Dilution"() -> (w4379:dbl)
            n3546 = local read "Synthesis/Name"() -> (w4381:string)
            n3547 = local read "Synthesis/Name"() -> (w4378:string)
            n3548 = local read "Synthesis/InjTemp"() -> (w4377:dbl)
            n3549 = local read "SampleOf"() -> (w4385:string)
            n3550 = local read "SampleGoal"() -> (w4375:string)
            n3551 = Bundle("Synthesis/InjTemp"=w4377, "Synthesis/Name"=w4378, "Synthesis/Dilution"=w4379, "Synthesis/DilutionPolyRatio"=w4380, "Synthesis/Name"=w4381, "Synthesis/Solvent"=w4382, "Synthesis/Polymer"=w4383, "Sample first cooldown"=w4384, "SampleOf"=w4385) -> (w4376:T2)  [unwired: 1 in]
            n3552 = local write "output cluster"(w4376) -> ()
            n3553 = call "SampleDetails.vi"("SampleDetailsClus"=w4376, "SampleGoal"=w4375, "Wrte to Obs"=TRUE ("NewSample in Obs"), "NewSampleDetails?"=TRUE, "Header?"=FALSE) -> ("SampleNameNoDate"=w4372:string, "SampleName"=w4373:string)
            n3554 = local write "Experiment Name"(w4372) -> ()
            n3555 = local write "Experiment Name With Date"(w4373) -> ()
          }
          event "Scan FSM Go to Cursor": Mouse Down {
            n3556 = event-data() -> ()  [unwired: 1 in, 8 out]
            n3557 = local write "Scan FSM Go to Cursor"(FALSE ("Scan FSM Go to Cursor")) -> ()
            n3558 = local read "NewDot"() -> (w4387:bool)
            n3559 = property on="XY Intensity Map" class="IntGraph (strict)"() -> ("Cursor.Cursor X"=w4388:dbl, "Cursor.Cursor Y"=w4389:dbl)  [unwired: 2 in, 2 out]
            n3560 = case shown="True" w4387 {
              frame False {
              }
              frame True {
                n3561 = local read "DotNum"() -> (w4391:dbl)
                n3562 = Increment(x=w4391) -> (x+1=w4390:dbl)
                n3563 = local write "DotNum"(w4390) -> ()
                n3564 = property on="DotNum" class="DigNum (strict)"("Val(Sgnl)"=w4390) -> ()  [unwired: 2 in, 2 out]
              }
            }
            n3565 = property on="FSM Y Axis Pos" class="DigNum (strict)"("Val(Sgnl)"=w4389) -> ()  [unwired: 2 in, 2 out]
            n3566 = property on="FSM X Axis Pos" class="DigNum (strict)"("Val(Sgnl)"=w4388) -> ()  [unwired: 2 in, 2 out]
          }
          event "DotNum": Value Change {
            w4395 = "\r"
            w4413 = "\r"
            w4401 = "%02d" ("format string")
            n3567 = event-data() -> ("NewVal"=w4403:dbl)  [unwired: 1 in, 5 out]
            n3568 = local read "Map Marker Y Pos"() -> (w4435:i8)
            n3569 = local read "Map Marker X Pos"() -> (w4436:i8)
            n3570 = local read "FSM Y Axis Pos"() -> (w4429:dbl)
            n3571 = Format Into String(w4436) -> (resulting string=w4434:string)  [unwired: 3 in, 1 out]
            n3572 = Format Into String(w4435) -> (resulting string=w4433:string)  [unwired: 3 in, 1 out]
            n3573 = local read "FSM X Axis Pos"() -> (w4428:dbl)
            n3574 = Format Into String(format string=w4401, initial string="#### NC" ("String"), w4403) -> (resulting string=w4406:string)  [unwired: 1 in, 1 out]
            n3575 = Format Into String(format string=w4401, initial string="NC", w4403) -> (resulting string=w4400:string)  [unwired: 1 in, 1 out]
            n3576 = Format Into String(format string="(%.2f,", initial string=" FSM ", w4428) -> (resulting string=w4425:string)  [unwired: 1 in, 1 out]
            n3577 = Format Into String(format string="%.2f)", w4429) -> (resulting string=w4423:string)  [unwired: 2 in, 1 out]
            n3578 = Concatenate Strings(w4400, "_Pos" ("string")) -> (w4404:string)
            n3579 = Concatenate Strings("\r", w4406, " @ " ("string"), w4434, "x" ("string"), w4433, w4425, "  " ("string"), w4423, w4413, "##### Position" ("string"), w4413) -> (w4397:string)
            n3580 = flat-sequence {
              tunnel: w4397 -> [w4444]
              tunnel: w4399 -> [w4447]
              tunnel: w4398 -> [w4446]
              tunnel: [w4445] -> w4392
              tunnel: w4393 -> [w4450]
              frame #0 {
                n3581 = call "Write2Markdown.vi"("String"=w4444) -> ()
              }
              frame #1 {
                n3582 = local read "ExportMapPosition?"() -> (w4445:bool)
                n3583 = case shown="True" w4445 {
                  tunnel: w4447 -> [_ w4449]
                  tunnel: w4446 -> [_ w4448]
                  frame False {
                  }
                  frame True {
                    n3584 = call <vilib>:"Write PNG File.vi"("image data"=w4449, "path to PNG file"=w4448) -> ()  [unwired: 8 in, 2 out]
                  }
                }
              }
              frame #2 {
                n3585 = call "Write2Markdown.vi"("String"=w4450) -> ()
              }
            }
            n3586 = invoke on="XY Intensity Map" class="IntGraph (strict)" method="Get Image"() -> ("image data"=w4399:T43)  [unwired: 6 in, 5 out]
            n3587 = Format Date/Time String(time format string (%c)="\\%Y-%m-%d_") -> (date/time string=w4419:string)  [unwired: 2 in]
            n3588 = Concatenate Strings(w4419, w4404, ".png" ("string")) -> (w4420:string)
            n3589 = Concatenate Strings("C:\\Users\\manip\\Documents\\CARODOT_Data\\doc\\CARODOC\\attachments", w4420) -> (w4418:string)
            n3590 = String To Path(string=w4418) -> (path=w4398:path)
            n3591 = Format Date/Time String(time format string (%c)="%Y-%m-%d_") -> (date/time string=w4412:string)  [unwired: 2 in]
            n3592 = Concatenate Strings(w4412, w4404, ".png" ("string")) -> (w4411:string)
            n3593 = Concatenate Strings("> ![\\|300](attachments/", w4411, ")", w4395) -> (w4394:string)
            n3594 = case shown="False" w4392 {
              tunnel: "##### Measurements" ("string") -> [w4439 w4443]
              tunnel: w4395 -> [w4438 w4442]
              tunnel: w4394 -> [_ w4441]
              tunnel: [w4437 w4440] -> w4393
              frame False {
                n3595 = Concatenate Strings(w4439, w4438) -> (w4437:string)
              }
              frame True {
                n3596 = Concatenate Strings(w4441, w4443, w4442) -> (w4440:string)
              }
            }
          }
          event "Scan FSM Set as Center": Value Change {
            n3597 = event-data() -> ("CtlRef"=w4464:refnum<vi>)  [unwired: 1 in, 5 out]
            n3598 = property class="Bool (strict)"(reference=w4464, "Value"=FALSE) -> ()  [unwired: 1 in, 2 out]
            n3599 = property on="XY Intensity Map" class="IntGraph (strict)"() -> ("Cursor.Cursor X"=w4454:dbl, "Cursor.Cursor Y"=w4452:dbl)  [unwired: 2 in, 2 out]
            n3600 = Multiply(x=w4454, y=1000.0) -> (x*y=w4461:dbl)
            n3601 = Multiply(x=w4452, y=1000.0) -> (x*y=w4456:dbl)
            n3602 = Round To Nearest(number=w4461) -> (nearest integer value=w4459:dbl)
            n3603 = Round To Nearest(number=w4456) -> (nearest integer value=w4458:dbl)
            n3604 = Divide(x=w4459, y=1000.0) -> (x/y=w4453:dbl)
            n3605 = Divide(x=w4458, y=1000.0) -> (x/y=w4451:dbl)
            n3606 = local write "Scan X Center (V)"(w4453) -> ()
            n3607 = local write "Scan Y Center (V)"(w4451) -> ()
          }
          event "Scan X Res. (V)", "Scan Y Res. (V)", "Scan X Tot. Length (V)", "Scan Y Tot. Length": Value Change {
            n3608 = event-data() -> ()  [unwired: 1 in, 6 out]
            n3609 = local read "Acq Time (ms)"() -> (w4468:dbl)
            n3610 = local read "Scan X Tot. Length (V)"() -> (w4479:dbl)
            n3611 = local read "Scan Y Res. (V)"() -> (w4475:dbl)
            n3612 = local read "Scan Y Tot. Length"() -> (w4474:dbl)
            n3613 = local read "Scan X Res. (V)"() -> (w4478:dbl)
            n3614 = Add(x=w4468, y=200.0) -> (x+y=w4466:dbl)
            n3615 = Divide(x=w4479, y=w4478) -> (x/y=w4477:dbl)
            n3616 = Divide(x=w4474, y=w4475) -> (x/y=w4476:dbl)
            n3617 = Divide(x=w4466, y=1000.0) -> (x/y=w4470:dbl)
            n3618 = Increment(x=w4477) -> (x+1=w4465:dbl)
            n3619 = Increment(x=w4476) -> (x+1=w4473:dbl)
            n3620 = local write "Scan Y Num. Pts"(w4473) -> ()
            n3621 = Multiply(x=w4465, y=w4473) -> (x*y=w4472:dbl)
            n3622 = local write "Scan X Num. Pts"(w4465) -> ()
            n3623 = Multiply(x=w4472, y=w4470) -> (x*y=w4469:dbl)
            n3624 = local write "Expected (s)"(w4469) -> ()
          }
          event "Shutter Ctrls", "KCubeSolenoidControl": Mouse Down {
            n3625 = event-data() -> ()  [unwired: 1 in, 8 out]
            n3626 = local read "KCube Shutter On?"() -> (w4480:bool)
            n3627 = control-ref of="Shutter Ctrls"() -> (w4482:refnum<vi>)
            n3628 = control-ref of="KCube Shutter Device Reference"() -> (w4481:refnum<vi>)
            n3629 = call "Shutter.vi"("KCube Shutter Device Reference 2"=w4481, "Shutter Ctrls 2"=w4482, "Shutter on?"=w4480) -> ()
          }
          event "Shutter Mode": Value Change {
            n3630 = event-data() -> ()  [unwired: 1 in, 6 out]
            n3631 = local read "KCube Shutter On?"() -> (w4483:bool)
            n3632 = case shown="True" w4483 {
              frame False {
              }
              frame True {
                # "1 Active == Laser on / Shutter off\n2 Inactive == Laser off / Shutter on\n\nThere are 4 operating modes for shutter:\n1 Manual\n2 Single Toggle\n3 Automatic Toggle\n4 Triggered"
                n3633 = local read "KCube Shutter Device Reference"() -> (w4485:refnum<k24>)
                n3634 = local read "Shutter Mode"() -> (w4484:i32)
                n3635 = invoke class="KCubeSolenoid" method="SetOperatingMode"(reference=w4485, "mode"=w4484) -> ()  [unwired: 2 in, 4 out]
              }
            }
          }
          event "Stop Everything & Quit?": Value Change {
            # "Stop program"
            n3636 = event-data() -> ("NewVal"=w4486:bool)  [unwired: 1 in, 5 out]
            "NewVal" <- w4486
          }
          event "TEC Output", "TEC Temperature", "Laser on? Control": Mouse Down; "Laser Diode Current Set": Value Change {
            # "Laser diode control"
            n3637 = event-data() -> ("CtlRef"=w4488:refnum<vi>)  [unwired: 1 in, 3 out]
            n3638 = local read "Laser Comm On?"() -> (w4487:bool)
            n3639 = case shown="True" w4487 {
              tunnel: w4488 -> [_ w4498]
              frame False {
              }
              frame True {
                n3640 = local read "Photodiode error out"() -> (w4497:errorcluster)
                n3641 = local read "Diode Driver Error"() -> (w4493:errorcluster)
                n3642 = local read "Photodiode handle out"() -> (w4496:refnum<visa-resource-name>)
                n3643 = property class="Ctl"(reference=w4498) -> ("Label.Text"=w4489:string)  [unwired: 1 in, 2 out]
                n3644 = local read "DDE"() -> (w4491:refnum<visa-resource-name>)
                n3645 = case shown="\"Laser on? Control\"" w4489 {
                  tunnel: w4491 -> [w4504 w4515 w4551 w4588 w4621]
                  tunnel: [w4503 w4514 w4550 w4590 w4621] -> w4494
                  tunnel: w4496 -> [w4501 w4510 w4549 w4591 w4620]
                  tunnel: w4497 -> [w4502 w4509 w4548 w4592 w4619]
                  tunnel: [w4501 w4506 w4547 w4591 w4620] -> w4495
                  tunnel: [w4502 w4511 w4546 w4592 w4619] -> w4490
                  tunnel: [w4500 w4508 w4545 w4589 w4618] -> w4492
                  tunnel: w4493 -> [w4499 w4507 w4544 w4587 w4618]
                  frame "TEC Temperature" {
                    n3646 = call <instrlib>:"TL4000 Measure Temperature.vi"("error in (no error)"=w4499, "instrument handle"=w4504) -> ("error out"=w4500:errorcluster, "Temperature"=w4505:dbl, "instrument handle out"=w4503:refnum<visa-resource-name>)  [unwired: 7 in]
                    n3647 = local write "TEC Temperature"(w4505) -> ()
                  }
                  frame "Laser on? Control" {
                    n3648 = flat-sequence {
                      tunnel: w4515 -> [w4523]
                      tunnel: [w4522] -> w4513
                      tunnel: [w4521] -> w4512
                      tunnel: w4507 -> [w4516]
                      tunnel: [w4534] -> w4514
                      tunnel: [w4535] -> w4508
                      tunnel: w4513 -> [w4535]
                      tunnel: w4512 -> [w4534]
                      tunnel: [w4533] -> w4506